vi "Dresden R2R Sputter 03.02.2018 IY24.vi"() -> ()   [LabVIEW 2009] (continued)
                        n3270 = local write "Pps_code_entry"("PF187=" ("Pps_code_entry")) -> ()
                      }
                      frame #1 {
                        n3271 = Wait (ms)(milliseconds to wait=u32 500) -> ()  [unwired: 1 out]
                      }
                      frame #2 {
                        n3272 = local write "Ppsok"(TRUE ("Ppsok")) -> ()
                      }
                    }
                  }
                }
              }
            }
            n3273 = case shown="True" w5019 {
              tunnel: w5023 -> [_ w5431]
              frame #0 {
              }
              frame #1 {
                n3274 = case shown="False" w5431 {
                  frame #0 {
                    n3275 = stacked-sequence {
                      frame #0 {
                        n3276 = local write "Pps_code_entry"("PF118=" ("Pps_code_entry")) -> ()
                      }
                      frame #1 {
                        n3277 = Wait (ms)(milliseconds to wait=u32 500) -> ()  [unwired: 1 out]
                      }
                      frame #2 {
                        n3278 = local write "Ppsok"(TRUE ("Ppsok")) -> ()
                      }
                    }
                  }
                  frame #1 {
                    n3279 = stacked-sequence {
                      frame #0 {
                        n3280 = local write "Pps_code_entry"("PF117=" ("Pps_code_entry")) -> ()
                      }
                      frame #1 {
                        n3281 = Wait (ms)(milliseconds to wait=u32 500) -> ()  [unwired: 1 out]
                      }
                      frame #2 {
                        n3282 = local write "Ppsok"(TRUE ("Ppsok")) -> ()
                      }
                    }
                  }
                }
              }
            }
            n3283 = case shown="True" w4829 {
              tunnel: w4833 -> [_ w5074]
              frame #0 {
              }
              frame #1 {
                n3284 = case shown="True" w5074 {
                  frame #0 {
                    n3285 = stacked-sequence {
                      frame #0 {
                        n3286 = local write "Pps_code_entry"("PF218=" ("Pps_code_entry")) -> ()
                      }
                      frame #1 {
                        n3287 = Wait (ms)(milliseconds to wait=u32 500) -> ()  [unwired: 1 out]
                      }
                      frame #2 {
                        n3288 = local write "Ppsok"(TRUE ("Ppsok")) -> ()
                      }
                    }
                  }
                  frame #1 {
                    n3289 = stacked-sequence {
                      frame #0 {
                        n3290 = local write "Pps_code_entry"("PF217=" ("Pps_code_entry")) -> ()
                      }
                      frame #1 {
                        n3291 = Wait (ms)(milliseconds to wait=u32 500) -> ()  [unwired: 1 out]
                      }
                      frame #2 {
                        n3292 = local write "Ppsok"(TRUE ("Ppsok")) -> ()
                      }
                    }
                  }
                }
              }
            }
            n3293 = case shown="True" w5059 {
              tunnel: w5063 -> [_ w5487]
              frame #0 {
              }
              frame #1 {
                n3294 = case shown="False" w5487 {
                  frame #0 {
                    n3295 = stacked-sequence {
                      frame #0 {
                        n3296 = local write "Pps_code_entry"("PF114=" ("Pps_code_entry")) -> ()
                      }
                      frame #1 {
                        n3297 = Wait (ms)(milliseconds to wait=u32 500) -> ()  [unwired: 1 out]
                      }
                      frame #2 {
                        n3298 = local write "Ppsok"(TRUE ("Ppsok")) -> ()
                      }
                    }
                  }
                  frame #1 {
                    n3299 = stacked-sequence {
                      frame #0 {
                        n3300 = local write "Pps_code_entry"("PF113=" ("Pps_code_entry")) -> ()
                      }
                      frame #1 {
                        n3301 = Wait (ms)(milliseconds to wait=u32 500) -> ()  [unwired: 1 out]
                      }
                      frame #2 {
                        n3302 = local write "Ppsok"(TRUE ("Ppsok")) -> ()
                      }
                    }
                  }
                }
              }
            }
            n3303 = case shown="True" w4989 {
              tunnel: w4993 -> [_ w5305]
              frame #0 {
              }
              frame #1 {
                n3304 = case shown="True" w5305 {
                  frame #0 {
                    n3305 = stacked-sequence {
                      frame #0 {
                        n3306 = local write "Pps_code_entry"("PF154=" ("Pps_code_entry")) -> ()
                      }
                      frame #1 {
                        n3307 = Wait (ms)(milliseconds to wait=u32 500) -> ()  [unwired: 1 out]
                      }
                      frame #2 {
                        n3308 = local write "Ppsok"(TRUE ("Ppsok")) -> ()
                      }
                    }
                  }
                  frame #1 {
                    n3309 = stacked-sequence {
                      frame #0 {
                        n3310 = local write "Pps_code_entry"("PF153=" ("Pps_code_entry")) -> ()
                      }
                      frame #1 {
                        n3311 = Wait (ms)(milliseconds to wait=u32 500) -> ()  [unwired: 1 out]
                      }
                      frame #2 {
                        n3312 = local write "Ppsok"(TRUE ("Ppsok")) -> ()
                      }
                    }
                  }
                }
              }
            }
            n3313 = case shown="True" w4888 {
              tunnel: w4884 -> [_ w5256]
              frame #0 {
              }
              frame #1 {
                n3314 = case shown="False" w5256 {
                  frame #0 {
                    n3315 = stacked-sequence {
                      frame #0 {
                        n3316 = local write "Pps_code_entry"("PF175=" ("Pps_code_entry")) -> ()
                      }
                      frame #1 {
                        n3317 = Wait (ms)(milliseconds to wait=u32 500) -> ()  [unwired: 1 out]
                      }
                      frame #2 {
                        n3318 = local write "Ppsok"(TRUE ("Ppsok")) -> ()
                      }
                    }
                  }
                  frame #1 {
                    n3319 = stacked-sequence {
                      frame #0 {
                        n3320 = local write "Pps_code_entry"("PF175=" ("Pps_code_entry")) -> ()
                      }
                      frame #1 {
                        n3321 = Wait (ms)(milliseconds to wait=u32 500) -> ()  [unwired: 1 out]
                      }
                      frame #2 {
                        n3322 = local write "Ppsok"(TRUE ("Ppsok")) -> ()
                      }
                    }
                  }
                }
              }
            }
            n3323 = case shown="True" w4913 {
              tunnel: w4909 -> [_ w5172]
              frame #0 {
              }
              frame #1 {
                n3324 = case shown="False" w5172 {
                  frame #0 {
                    n3325 = stacked-sequence {
                      frame #0 {
                        n3326 = local write "Pps_code_entry"("PF186=" ("Pps_code_entry")) -> ()
                      }
                      frame #1 {
                        n3327 = Wait (ms)(milliseconds to wait=u32 500) -> ()  [unwired: 1 out]
                      }
                      frame #2 {
                        n3328 = local write "Ppsok"(TRUE ("Ppsok")) -> ()
                      }
                    }
                  }
                  frame #1 {
                    n3329 = stacked-sequence {
                      frame #0 {
                        n3330 = local write "Pps_code_entry"("PF185=" ("Pps_code_entry")) -> ()
                      }
                      frame #1 {
                        n3331 = Wait (ms)(milliseconds to wait=u32 500) -> ()  [unwired: 1 out]
                      }
                      frame #2 {
                        n3332 = local write "Ppsok"(TRUE ("Ppsok")) -> ()
                      }
                    }
                  }
                }
              }
            }
            n3333 = case shown="True" w4868 {
              tunnel: w4864 -> [_ w5228]
              frame #0 {
              }
              frame #1 {
                n3334 = case shown="False" w5228 {
                  frame #0 {
                    n3335 = stacked-sequence {
                      frame #0 {
                        n3336 = local write "Pps_code_entry"("PF180=" ("Pps_code_entry")) -> ()
                      }
                      frame #1 {
                        n3337 = Wait (ms)(milliseconds to wait=u32 500) -> ()  [unwired: 1 out]
                      }
                      frame #2 {
                        n3338 = local write "Ppsok"(TRUE ("Ppsok")) -> ()
                      }
                    }
                  }
                  frame #1 {
                    n3339 = stacked-sequence {
                      frame #0 {
                        n3340 = local write "Pps_code_entry"("PF179=" ("Pps_code_entry")) -> ()
                      }
                      frame #1 {
                        n3341 = Wait (ms)(milliseconds to wait=u32 500) -> ()  [unwired: 1 out]
                      }
                      frame #2 {
                        n3342 = local write "Ppsok"(TRUE ("Ppsok")) -> ()
                      }
                    }
                  }
                }
              }
            }
            n3343 = case shown="True" w4779 {
              tunnel: w4783 -> [_ w5144]
              frame #0 {
              }
              frame #1 {
                n3344 = case shown="False" w5144 {
                  frame #0 {
                    n3345 = stacked-sequence {
                      frame #0 {
                        n3346 = local write "Pps_code_entry"("PF210=" ("Pps_code_entry")) -> ()
                      }
                      frame #1 {
                        n3347 = Wait (ms)(milliseconds to wait=u32 500) -> ()  [unwired: 1 out]
                      }
                      frame #2 {
                        n3348 = local write "Ppsok"(TRUE ("Ppsok")) -> ()
                      }
                    }
                  }
                  frame #1 {
                    n3349 = stacked-sequence {
                      frame #0 {
                        n3350 = local write "Pps_code_entry"("PF209=" ("Pps_code_entry")) -> ()
                      }
                      frame #1 {
                        n3351 = Wait (ms)(milliseconds to wait=u32 500) -> ()  [unwired: 1 out]
                      }
                      frame #2 {
                        n3352 = local write "Ppsok"(TRUE ("Ppsok")) -> ()
                      }
                    }
                  }
                }
              }
            }
            n3353 = case shown="True" w5008 {
              tunnel: w5004 -> [_ w5410]
              frame #0 {
              }
              frame #1 {
                n3354 = case shown="False" w5410 {
                  frame #0 {
                    n3355 = stacked-sequence {
                      frame #0 {
                        n3356 = local write "Pps_code_entry"("PF120=" ("Pps_code_entry")) -> ()
                      }
                      frame #1 {
                        n3357 = Wait (ms)(milliseconds to wait=u32 500) -> ()  [unwired: 1 out]
                      }
                      frame #2 {
                        n3358 = local write "Ppsok"(TRUE ("Ppsok")) -> ()
                      }
                    }
                  }
                  frame #1 {
                    n3359 = stacked-sequence {
                      frame #0 {
                        n3360 = local write "Pps_code_entry"("PF119=" ("Pps_code_entry")) -> ()
                      }
                      frame #1 {
                        n3361 = Wait (ms)(milliseconds to wait=u32 500) -> ()  [unwired: 1 out]
                      }
                      frame #2 {
                        n3362 = local write "Ppsok"(TRUE ("Ppsok")) -> ()
                      }
                    }
                  }
                }
              }
            }
            n3363 = case shown="True" w4939 {
              tunnel: w4943 -> [_ w5375]
              frame #0 {
              }
              frame #1 {
                n3364 = case shown="True" w5375 {
                  frame #0 {
                    n3365 = stacked-sequence {
                      frame #0 {
                        n3366 = local write "Pps_code_entry"("PF142=" ("Pps_code_entry")) -> ()
                      }
                      frame #1 {
                        n3367 = Wait (ms)(milliseconds to wait=u32 500) -> ()  [unwired: 1 out]
                      }
                      frame #2 {
                        n3368 = local write "Ppsok"(TRUE ("Ppsok")) -> ()
                      }
                    }
                  }
                  frame #1 {
                    n3369 = stacked-sequence {
                      frame #0 {
                        n3370 = local write "Pps_code_entry"("PF141=" ("Pps_code_entry")) -> ()
                      }
                      frame #1 {
                        n3371 = Wait (ms)(milliseconds to wait=u32 500) -> ()  [unwired: 1 out]
                      }
                      frame #2 {
                        n3372 = local write "Ppsok"(TRUE ("Ppsok")) -> ()
                      }
                    }
                  }
                }
              }
            }
            n3373 = case shown="True" w4914 {
              tunnel: w4918 -> [_ w5284]
              frame #0 {
              }
              frame #1 {
                n3374 = case shown="False" w5284 {
                  frame #0 {
                    n3375 = stacked-sequence {
                      frame #0 {
                        n3376 = local write "Pps_code_entry"("PF152=" ("Pps_code_entry")) -> ()
                      }
                      frame #1 {
                        n3377 = Wait (ms)(milliseconds to wait=u32 500) -> ()  [unwired: 1 out]
                      }
                      frame #2 {
                        n3378 = local write "Ppsok"(TRUE ("Ppsok")) -> ()
                      }
                    }
                  }
                  frame #1 {
                    n3379 = stacked-sequence {
                      frame #0 {
                        n3380 = local write "Pps_code_entry"("PF151=" ("Pps_code_entry")) -> ()
                      }
                      frame #1 {
                        n3381 = Wait (ms)(milliseconds to wait=u32 500) -> ()  [unwired: 1 out]
                      }
                      frame #2 {
                        n3382 = local write "Ppsok"(TRUE ("Ppsok")) -> ()
                      }
                    }
                  }
                }
              }
            }
            n3383 = case shown="True" w4799 {
              tunnel: w4803 -> [_ w5116]
              frame #0 {
              }
              frame #1 {
                n3384 = case shown="True" w5116 {
                  frame #0 {
                    n3385 = stacked-sequence {
                      frame #0 {
                        n3386 = local write "Pps_code_entry"("PF214=" ("Pps_code_entry")) -> ()
                      }
                      frame #1 {
                        n3387 = Wait (ms)(milliseconds to wait=u32 500) -> ()  [unwired: 1 out]
                      }
                      frame #2 {
                        n3388 = local write "Ppsok"(TRUE ("Ppsok")) -> ()
                      }
                    }
                  }
                  frame #1 {
                    n3389 = stacked-sequence {
                      frame #0 {
                        n3390 = local write "Pps_code_entry"("PF213=" ("Pps_code_entry")) -> ()
                      }
                      frame #1 {
                        n3391 = Wait (ms)(milliseconds to wait=u32 500) -> ()  [unwired: 1 out]
                      }
                      frame #2 {
                        n3392 = local write "Ppsok"(TRUE ("Ppsok")) -> ()
                      }
                    }
                  }
                }
              }
            }
            n3393 = case shown="True" w4959 {
              tunnel: w4963 -> [_ w5347]
              frame #0 {
              }
              frame #1 {
                n3394 = case shown="True" w5347 {
                  frame #0 {
                    n3395 = stacked-sequence {
                      frame #0 {
                        n3396 = local write "Pps_code_entry"("PF146=" ("Pps_code_entry")) -> ()
                      }
                      frame #1 {
                        n3397 = Wait (ms)(milliseconds to wait=u32 500) -> ()  [unwired: 1 out]
                      }
                      frame #2 {
                        n3398 = local write "Ppsok"(TRUE ("Ppsok")) -> ()
                      }
                    }
                  }
                  frame #1 {
                    n3399 = stacked-sequence {
                      frame #0 {
                        n3400 = local write "Pps_code_entry"("PF145=" ("Pps_code_entry")) -> ()
                      }
                      frame #1 {
                        n3401 = Wait (ms)(milliseconds to wait=u32 500) -> ()  [unwired: 1 out]
                      }
                      frame #2 {
                        n3402 = local write "Ppsok"(TRUE ("Ppsok")) -> ()
                      }
                    }
                  }
                }
              }
            }
            n3403 = case shown="True" w5058 {
              tunnel: w5054 -> [_ w5480]
              frame #0 {
              }
              frame #1 {
                n3404 = case shown="False" w5480 {
                  frame #0 {
                    n3405 = stacked-sequence {
                      frame #0 {
                        n3406 = local write "Pps_code_entry"("PF112=" ("Pps_code_entry")) -> ()
                      }
                      frame #1 {
                        n3407 = Wait (ms)(milliseconds to wait=u32 500) -> ()  [unwired: 1 out]
                      }
                      frame #2 {
                        n3408 = local write "Ppsok"(TRUE ("Ppsok")) -> ()
                      }
                    }
                  }
                  frame #1 {
                    n3409 = stacked-sequence {
                      frame #0 {
                        n3410 = local write "Pps_code_entry"("PF111=" ("Pps_code_entry")) -> ()
                      }
                      frame #1 {
                        n3411 = Wait (ms)(milliseconds to wait=u32 500) -> ()  [unwired: 1 out]
                      }
                      frame #2 {
                        n3412 = local write "Ppsok"(TRUE ("Ppsok")) -> ()
                      }
                    }
                  }
                }
              }
            }
            n3413 = case shown="True" w5038 {
              tunnel: w5034 -> [_ w5452]
              frame #0 {
              }
              frame #1 {
                n3414 = case shown="False" w5452 {
                  frame #0 {
                    n3415 = stacked-sequence {
                      frame #0 {
                        n3416 = local write "Pps_code_entry"("PF116=" ("Pps_code_entry")) -> ()
                      }
                      frame #1 {
                        n3417 = Wait (ms)(milliseconds to wait=u32 500) -> ()  [unwired: 1 out]
                      }
                      frame #2 {
                        n3418 = local write "Ppsok"(TRUE ("Ppsok")) -> ()
                      }
                    }
                  }
                  frame #1 {
                    n3419 = stacked-sequence {
                      frame #0 {
                        n3420 = local write "Pps_code_entry"("PF115=" ("Pps_code_entry")) -> ()
                      }
                      frame #1 {
                        n3421 = Wait (ms)(milliseconds to wait=u32 500) -> ()  [unwired: 1 out]
                      }
                      frame #2 {
                        n3422 = local write "Ppsok"(TRUE ("Ppsok")) -> ()
                      }
                    }
                  }
                }
              }
            }
            n3423 = local read "Trns_gv_2_3_on"() -> (w4994:bool)
            n3424 = local read "Ch3_Bg_bv_on"() -> (w4844:bool)
            n3425 = local read "Trns_gv_1_2_on"() -> (w5003:bool)
            n3426 = local read "Ch4_Bg_bv_on"() -> (w4823:bool)
            n3427 = local read "Ch2_Bg_bv_on"() -> (w4983:bool)
            n3428 = local read "Ch3_Ch_atm_on"() -> (w4879:bool)
            n3429 = local read "Ch4_Ch_atm_on"() -> (w4788:bool)
            n3430 = local read "Ch2_Ch_atm_on"() -> (w4948:bool)
            n3431 = local read "Ch1_Bg_bv_on"() -> (w5014:bool)
            n3432 = local read "Ch3_Ch_cc_on"() -> (w4878:bool)
            n3433 = local read "Ch4_Ch_cc_on"() -> (w4789:bool)
            n3434 = local read "Ch1_Ch_atm_on"() -> (w5049:bool)
            n3435 = local read "Ch2_Ch_cc_on"() -> (w4949:bool)
            n3436 = local read "Ch1_Ch_cc_on"() -> (w5048:bool)
            n3437 = local read "Ch3_Ch_pg_on"() -> (w4863:bool)
            n3438 = local read "Ch4_Ch_pg_on"() -> (w4804:bool)
            n3439 = local read "Ch2_Ch_pg_on"() -> (w4964:bool)
            n3440 = local read "Ch1_Ch_pg_on"() -> (w5033:bool)
            n3441 = feedback #98() -> (w4862:bool)  [unwired: 1 in]
            n3442 = feedback #99() -> (w4845:bool)  [unwired: 1 in]
            n3443 = feedback #100() -> (w4995:bool)  [unwired: 1 in]
            n3444 = feedback #101() -> (w4805:bool)  [unwired: 1 in]
            n3445 = feedback #102() -> (w4822:bool)  [unwired: 1 in]
            n3446 = feedback #103() -> (w4965:bool)  [unwired: 1 in]
            n3447 = feedback #104() -> (w4982:bool)  [unwired: 1 in]
            n3448 = feedback #105() -> (w5002:bool)  [unwired: 1 in]
            n3449 = feedback #106() -> (w5032:bool)  [unwired: 1 in]
            n3450 = feedback #107() -> (w5015:bool)  [unwired: 1 in]
            n3451 = feedback #108() -> (w4877:bool)  [unwired: 1 in]
            n3452 = feedback #109() -> (w4790:bool)  [unwired: 1 in]
            n3453 = feedback #110() -> (w4950:bool)  [unwired: 1 in]
            n3454 = feedback #111() -> (w4880:bool)  [unwired: 1 in]
            n3455 = feedback #112() -> (w4787:bool)  [unwired: 1 in]
            n3456 = feedback #113() -> (w4947:bool)  [unwired: 1 in]
            n3457 = feedback #114() -> (w5047:bool)  [unwired: 1 in]
            n3458 = feedback #115() -> (w5050:bool)  [unwired: 1 in]
            n3459 = Boolean To (0,1)(Boolean=w4863) -> (0, 1=w4861:i16)
            n3460 = Boolean To (0,1)(Boolean=w4862) -> (0, 1=w4860:i16)
            n3461 = Boolean To (0,1)(Boolean=w4844) -> (0, 1=w4846:i16)
            n3462 = Boolean To (0,1)(Boolean=w4845) -> (0, 1=w4847:i16)
            n3463 = Boolean To (0,1)(Boolean=w4994) -> (0, 1=w4996:i16)
            n3464 = Boolean To (0,1)(Boolean=w4995) -> (0, 1=w4997:i16)
            n3465 = Boolean To (0,1)(Boolean=w4804) -> (0, 1=w4806:i16)
            n3466 = Boolean To (0,1)(Boolean=w4805) -> (0, 1=w4807:i16)
            n3467 = Boolean To (0,1)(Boolean=w4823) -> (0, 1=w4821:i16)
            n3468 = Boolean To (0,1)(Boolean=w4822) -> (0, 1=w4820:i16)
            n3469 = Boolean To (0,1)(Boolean=w4964) -> (0, 1=w4966:i16)
            n3470 = Boolean To (0,1)(Boolean=w4965) -> (0, 1=w4967:i16)
            n3471 = Boolean To (0,1)(Boolean=w4983) -> (0, 1=w4981:i16)
            n3472 = Boolean To (0,1)(Boolean=w4982) -> (0, 1=w4980:i16)
            n3473 = Boolean To (0,1)(Boolean=w5003) -> (0, 1=w5001:i16)
            n3474 = Boolean To (0,1)(Boolean=w5002) -> (0, 1=w5000:i16)
            n3475 = Boolean To (0,1)(Boolean=w5033) -> (0, 1=w5031:i16)
            n3476 = Boolean To (0,1)(Boolean=w5032) -> (0, 1=w5030:i16)
            n3477 = Boolean To (0,1)(Boolean=w5014) -> (0, 1=w5016:i16)
            n3478 = Boolean To (0,1)(Boolean=w5015) -> (0, 1=w5017:i16)
            n3479 = Boolean To (0,1)(Boolean=w4878) -> (0, 1=w4876:i16)
            n3480 = Boolean To (0,1)(Boolean=w4877) -> (0, 1=w4875:i16)
            n3481 = Boolean To (0,1)(Boolean=w4789) -> (0, 1=w4791:i16)
            n3482 = Boolean To (0,1)(Boolean=w4790) -> (0, 1=w4792:i16)
            n3483 = Boolean To (0,1)(Boolean=w4949) -> (0, 1=w4951:i16)
            n3484 = Boolean To (0,1)(Boolean=w4950) -> (0, 1=w4952:i16)
            n3485 = Boolean To (0,1)(Boolean=w4879) -> (0, 1=w4881:i16)
            n3486 = Boolean To (0,1)(Boolean=w4880) -> (0, 1=w4882:i16)
            n3487 = Boolean To (0,1)(Boolean=w4788) -> (0, 1=w4786:i16)
            n3488 = Boolean To (0,1)(Boolean=w4787) -> (0, 1=w4785:i16)
            n3489 = Boolean To (0,1)(Boolean=w4948) -> (0, 1=w4946:i16)
            n3490 = Boolean To (0,1)(Boolean=w4947) -> (0, 1=w4945:i16)
            n3491 = Boolean To (0,1)(Boolean=w5048) -> (0, 1=w5046:i16)
            n3492 = Boolean To (0,1)(Boolean=w5047) -> (0, 1=w5045:i16)
            n3493 = Boolean To (0,1)(Boolean=w5049) -> (0, 1=w5051:i16)
            n3494 = Boolean To (0,1)(Boolean=w5050) -> (0, 1=w5052:i16)
            n3495 = Not Equal?(x=w4861, y=w4860) -> (x != y?=w4859:bool)
            n3496 = Not Equal?(x=w4846, y=w4847) -> (x != y?=w4848:bool)
            n3497 = Not Equal?(x=w4996, y=w4997) -> (x != y?=w4998:bool)
            n3498 = Not Equal?(x=w4806, y=w4807) -> (x != y?=w4808:bool)
            n3499 = Not Equal?(x=w4821, y=w4820) -> (x != y?=w4819:bool)
            n3500 = Not Equal?(x=w4966, y=w4967) -> (x != y?=w4968:bool)
            n3501 = Not Equal?(x=w4981, y=w4980) -> (x != y?=w4979:bool)
            n3502 = Not Equal?(x=w5001, y=w5000) -> (x != y?=w4999:bool)
            n3503 = Not Equal?(x=w5031, y=w5030) -> (x != y?=w5029:bool)
            n3504 = Not Equal?(x=w5016, y=w5017) -> (x != y?=w5018:bool)
            n3505 = Not Equal?(x=w4876, y=w4875) -> (x != y?=w4874:bool)
            n3506 = Not Equal?(x=w4791, y=w4792) -> (x != y?=w4793:bool)
            n3507 = Not Equal?(x=w4951, y=w4952) -> (x != y?=w4953:bool)
            n3508 = Not Equal?(x=w4881, y=w4882) -> (x != y?=w4883:bool)
            n3509 = Not Equal?(x=w4786, y=w4785) -> (x != y?=w4784:bool)
            n3510 = Not Equal?(x=w4946, y=w4945) -> (x != y?=w4944:bool)
            n3511 = Not Equal?(x=w5046, y=w5045) -> (x != y?=w5044:bool)
            n3512 = Not Equal?(x=w5051, y=w5052) -> (x != y?=w5053:bool)
            n3513 = case shown="True" w4859 {
              tunnel: w4863 -> [_ w5221]
              frame #0 {
              }
              frame #1 {
                n3514 = case shown="True" w5221 {
                  frame #0 {
                    n3515 = stacked-sequence {
                      frame #0 {
                        n3516 = local write "Pps_code_entry"("PF194=" ("Pps_code_entry")) -> ()
                      }
                      frame #1 {
                        n3517 = Wait (ms)(milliseconds to wait=u32 500) -> ()  [unwired: 1 out]
                      }
                      frame #2 {
                        n3518 = local write "Ppsok"(TRUE ("Ppsok")) -> ()
                      }
                    }
                  }
                  frame #1 {
                    n3519 = stacked-sequence {
                      frame #0 {
                        n3520 = local write "Pps_code_entry"("PF193=" ("Pps_code_entry")) -> ()
                      }
                      frame #1 {
                        n3521 = Wait (ms)(milliseconds to wait=u32 500) -> ()  [unwired: 1 out]
                      }
                      frame #2 {
                        n3522 = local write "Ppsok"(TRUE ("Ppsok")) -> ()
                      }
                    }
                  }
                }
              }
            }
            n3523 = case shown="True" w4848 {
              tunnel: w4844 -> [_ w5200]
              frame #0 {
              }
              frame #1 {
                n3524 = case shown="True" w5200 {
                  frame #0 {
                    n3525 = stacked-sequence {
                      frame #0 {
                        n3526 = local write "Pps_code_entry"("PF196=" ("Pps_code_entry")) -> ()
                      }
                      frame #1 {
                        n3527 = Wait (ms)(milliseconds to wait=u32 500) -> ()  [unwired: 1 out]
                      }
                      frame #2 {
                        n3528 = local write "Ppsok"(TRUE ("Ppsok")) -> ()
                      }
                    }
                  }
                  frame #1 {
                    n3529 = stacked-sequence {
                      frame #0 {
                        n3530 = local write "Pps_code_entry"("PF195=" ("Pps_code_entry")) -> ()
                      }
                      frame #1 {
                        n3531 = Wait (ms)(milliseconds to wait=u32 500) -> ()  [unwired: 1 out]
                      }
                      frame #2 {
                        n3532 = local write "Ppsok"(TRUE ("Ppsok")) -> ()
                      }
                    }
                  }
                }
              }
            }
            n3533 = case shown="True" w4998 {
              tunnel: w4994 -> [_ w5298]
              frame #0 {
              }
              frame #1 {
                n3534 = case shown="False" w5298 {
                  frame #0 {
                    n3535 = stacked-sequence {
                      frame #0 {
                        n3536 = local write "Pps_code_entry"("PF164=" ("Pps_code_entry")) -> ()
                      }
                      frame #1 {
                        n3537 = Wait (ms)(milliseconds to wait=u32 500) -> ()  [unwired: 1 out]
                      }
                      frame #2 {
                        n3538 = local write "Ppsok"(TRUE ("Ppsok")) -> ()
                      }
                    }
                  }
                  frame #1 {
                    n3539 = stacked-sequence {
                      frame #0 {
                        n3540 = local write "Pps_code_entry"("PF163=" ("Pps_code_entry")) -> ()
                      }
                      frame #1 {
                        n3541 = Wait (ms)(milliseconds to wait=u32 500) -> ()  [unwired: 1 out]
                      }
                      frame #2 {
                        n3542 = local write "Ppsok"(TRUE ("Ppsok")) -> ()
                      }
                    }
                  }
                }
              }
            }
            n3543 = case shown="True" w4808 {
              tunnel: w4804 -> [_ w5109]
              frame #0 {
              }
              frame #1 {
                n3544 = case shown="True" w5109 {
                  frame #0 {
                    n3545 = stacked-sequence {
                      frame #0 {
                        n3546 = local write "Pps_code_entry"("PF224=" ("Pps_code_entry")) -> ()
                      }
                      frame #1 {
                        n3547 = Wait (ms)(milliseconds to wait=u32 500) -> ()  [unwired: 1 out]
                      }
                      frame #2 {
                        n3548 = local write "Ppsok"(TRUE ("Ppsok")) -> ()
                      }
                    }
                  }
                  frame #1 {
                    n3549 = stacked-sequence {
                      frame #0 {
                        n3550 = local write "Pps_code_entry"("PF223=" ("Pps_code_entry")) -> ()
                      }
                      frame #1 {
                        n3551 = Wait (ms)(milliseconds to wait=u32 500) -> ()  [unwired: 1 out]
                      }
                      frame #2 {
                        n3552 = local write "Ppsok"(TRUE ("Ppsok")) -> ()
                      }
                    }
                  }
                }
              }
            }
            n3553 = case shown="True" w4819 {
              tunnel: w4823 -> [_ w5088]
              frame #0 {
              }
              frame #1 {
                n3554 = case shown="False" w5088 {
                  frame #0 {
                    n3555 = stacked-sequence {
                      frame #0 {
                        n3556 = local write "Pps_code_entry"("PF226=" ("Pps_code_entry")) -> ()
                      }
                      frame #1 {
                        n3557 = Wait (ms)(milliseconds to wait=u32 500) -> ()  [unwired: 1 out]
                      }
                      frame #2 {
                        n3558 = local write "Ppsok"(TRUE ("Ppsok")) -> ()
                      }
                    }
                  }
                  frame #1 {
                    n3559 = stacked-sequence {
                      frame #0 {
                        n3560 = local write "Pps_code_entry"("PF225=" ("Pps_code_entry")) -> ()
                      }
                      frame #1 {
                        n3561 = Wait (ms)(milliseconds to wait=u32 500) -> ()  [unwired: 1 out]
                      }
                      frame #2 {
                        n3562 = local write "Ppsok"(TRUE ("Ppsok")) -> ()
                      }
                    }
                  }
                }
              }
            }
            n3563 = case shown="True" w4968 {
              tunnel: w4964 -> [_ w5340]
              frame #0 {
              }
              frame #1 {
                n3564 = case shown="True" w5340 {
                  frame #0 {
                    n3565 = stacked-sequence {
                      frame #0 {
                        n3566 = local write "Pps_code_entry"("PF160=" ("Pps_code_entry")) -> ()
                      }
                      frame #1 {
                        n3567 = Wait (ms)(milliseconds to wait=u32 500) -> ()  [unwired: 1 out]
                      }
                      frame #2 {
                        n3568 = local write "Ppsok"(TRUE ("Ppsok")) -> ()
                      }
                    }
                  }
                  frame #1 {
                    n3569 = stacked-sequence {
                      frame #0 {
                        n3570 = local write "Pps_code_entry"("PF159=" ("Pps_code_entry")) -> ()
                      }
                      frame #1 {
                        n3571 = Wait (ms)(milliseconds to wait=u32 500) -> ()  [unwired: 1 out]
                      }
                      frame #2 {
                        n3572 = local write "Ppsok"(TRUE ("Ppsok")) -> ()
                      }
                    }
                  }
                }
              }
            }
            n3573 = case shown="True" w4979 {
              tunnel: w4983 -> [_ w5319]
              frame #0 {
              }
              frame #1 {
                n3574 = case shown="False" w5319 {
                  frame #0 {
                    n3575 = stacked-sequence {
                      frame #0 {
                        n3576 = local write "Pps_code_entry"("PF162=" ("Pps_code_entry")) -> ()
                      }
                      frame #1 {
                        n3577 = Wait (ms)(milliseconds to wait=u32 500) -> ()  [unwired: 1 out]
                      }
                      frame #2 {
                        n3578 = local write "Ppsok"(TRUE ("Ppsok")) -> ()
                      }
                    }
                  }
                  frame #1 {
                    n3579 = stacked-sequence {
                      frame #0 {
                        n3580 = local write "Pps_code_entry"("PF161=" ("Pps_code_entry")) -> ()
                      }
                      frame #1 {
                        n3581 = Wait (ms)(milliseconds to wait=u32 500) -> ()  [unwired: 1 out]
                      }
                      frame #2 {
                        n3582 = local write "Ppsok"(TRUE ("Ppsok")) -> ()
                      }
                    }
                  }
                }
              }
            }
            n3583 = case shown="True" w4999 {
              tunnel: w5003 -> [_ w5403]
              frame #0 {
              }
              frame #1 {
                n3584 = case shown="True" w5403 {
                  frame #0 {
                    n3585 = stacked-sequence {
                      frame #0 {
                        n3586 = local write "Pps_code_entry"("PF130=" ("Pps_code_entry")) -> ()
                      }
                      frame #1 {
                        n3587 = Wait (ms)(milliseconds to wait=u32 500) -> ()  [unwired: 1 out]
                      }
                      frame #2 {
                        n3588 = local write "Ppsok"(TRUE ("Ppsok")) -> ()
                      }
                    }
                  }
                  frame #1 {
                    n3589 = stacked-sequence {
                      frame #0 {
                        n3590 = local write "Pps_code_entry"("PF129=" ("Pps_code_entry")) -> ()
                      }
                      frame #1 {
                        n3591 = Wait (ms)(milliseconds to wait=u32 500) -> ()  [unwired: 1 out]
                      }
                      frame #2 {
                        n3592 = local write "Ppsok"(TRUE ("Ppsok")) -> ()
                      }
                    }
                  }
                }
              }
            }
            n3593 = case shown="True" w5029 {
              tunnel: w5033 -> [_ w5445]
              frame #0 {
              }
              frame #1 {
                n3594 = case shown="False" w5445 {
                  frame #0 {
                    n3595 = stacked-sequence {
                      frame #0 {
                        n3596 = local write "Pps_code_entry"("PF126=" ("Pps_code_entry")) -> ()
                      }
                      frame #1 {
                        n3597 = Wait (ms)(milliseconds to wait=u32 500) -> ()  [unwired: 1 out]
                      }
                      frame #2 {
                        n3598 = local write "Ppsok"(TRUE ("Ppsok")) -> ()
                      }
                    }
                  }
                  frame #1 {
                    n3599 = stacked-sequence {
                      frame #0 {
                        n3600 = local write "Pps_code_entry"("PF125=" ("Pps_code_entry")) -> ()
                      }
                      frame #1 {
                        n3601 = Wait (ms)(milliseconds to wait=u32 500) -> ()  [unwired: 1 out]
                      }
                      frame #2 {
                        n3602 = local write "Ppsok"(TRUE ("Ppsok")) -> ()
                      }
                    }
                  }
                }
              }
            }
            n3603 = case shown="True" w5018 {
              tunnel: w5014 -> [_ w5424]
              frame #0 {
              }
              frame #1 {
                n3604 = case shown="True" w5424 {
                  frame #0 {
                    n3605 = stacked-sequence {
                      frame #0 {
                        n3606 = local write "Pps_code_entry"("PF128=" ("Pps_code_entry")) -> ()
                      }
                      frame #1 {
                        n3607 = Wait (ms)(milliseconds to wait=u32 500) -> ()  [unwired: 1 out]
                      }
                      frame #2 {
                        n3608 = local write "Ppsok"(TRUE ("Ppsok")) -> ()
                      }
                    }
                  }
                  frame #1 {
                    n3609 = stacked-sequence {
                      frame #0 {
                        n3610 = local write "Pps_code_entry"("PF127=" ("Pps_code_entry")) -> ()
                      }
                      frame #1 {
                        n3611 = Wait (ms)(milliseconds to wait=u32 500) -> ()  [unwired: 1 out]
                      }
                      frame #2 {
                        n3612 = local write "Ppsok"(TRUE ("Ppsok")) -> ()
                      }
                    }
                  }
                }
              }
            }
            n3613 = case shown="True" w4874 {
              tunnel: w4878 -> [_ w5242]
              frame #0 {
              }
              frame #1 {
                n3614 = case shown="False" w5242 {
                  frame #0 {
                    n3615 = stacked-sequence {
                      frame #0 {
                        n3616 = local write "Pps_code_entry"("PF192=" ("Pps_code_entry")) -> ()
                      }
                      frame #1 {
                        n3617 = Wait (ms)(milliseconds to wait=u32 500) -> ()  [unwired: 1 out]
                      }
                      frame #2 {
                        n3618 = local write "Ppsok"(TRUE ("Ppsok")) -> ()
                      }
                    }
                  }
                  frame #1 {
                    n3619 = stacked-sequence {
                      frame #0 {
                        n3620 = local write "Pps_code_entry"("PF191=" ("Pps_code_entry")) -> ()
                      }
                      frame #1 {
                        n3621 = Wait (ms)(milliseconds to wait=u32 500) -> ()  [unwired: 1 out]
                      }
                      frame #2 {
                        n3622 = local write "Ppsok"(TRUE ("Ppsok")) -> ()
                      }
                    }
                  }
                }
              }
            }
            n3623 = case shown="True" w4793 {
              tunnel: w4789 -> [_ w5130]
              frame #0 {
              }
              frame #1 {
                n3624 = case shown="False" w5130 {
                  frame #0 {
                    n3625 = stacked-sequence {
                      frame #0 {
                        n3626 = local write "Pps_code_entry"("PF222=" ("Pps_code_entry")) -> ()
                      }
                      frame #1 {
                        n3627 = Wait (ms)(milliseconds to wait=u32 500) -> ()  [unwired: 1 out]
                      }
                      frame #2 {
                        n3628 = local write "Ppsok"(TRUE ("Ppsok")) -> ()
                      }
                    }
                  }
                  frame #1 {
                    n3629 = stacked-sequence {
                      frame #0 {
                        n3630 = local write "Pps_code_entry"("PF221=" ("Pps_code_entry")) -> ()
                      }
                      frame #1 {
                        n3631 = Wait (ms)(milliseconds to wait=u32 500) -> ()  [unwired: 1 out]
                      }
                      frame #2 {
                        n3632 = local write "Ppsok"(TRUE ("Ppsok")) -> ()
                      }
                    }
                  }
                }
              }
            }
            n3633 = case shown="True" w4953 {
              tunnel: w4949 -> [_ w5361]
              frame #0 {
              }
              frame #1 {
                n3634 = case shown="True" w5361 {
                  frame #0 {
                    n3635 = stacked-sequence {
                      frame #0 {
                        n3636 = local write "Pps_code_entry"("PF158=" ("Pps_code_entry")) -> ()
                      }
                      frame #1 {
                        n3637 = Wait (ms)(milliseconds to wait=u32 500) -> ()  [unwired: 1 out]
                      }
                      frame #2 {
                        n3638 = local write "Ppsok"(TRUE ("Ppsok")) -> ()
                      }
                    }
                  }
                  frame #1 {
                    n3639 = stacked-sequence {
                      frame #0 {
                        n3640 = local write "Pps_code_entry"("PF157=" ("Pps_code_entry")) -> ()
                      }
                      frame #1 {
                        n3641 = Wait (ms)(milliseconds to wait=u32 500) -> ()  [unwired: 1 out]
                      }
                      frame #2 {
                        n3642 = local write "Ppsok"(TRUE ("Ppsok")) -> ()
                      }
                    }
                  }
                }
              }
            }
            n3643 = case shown="True" w4883 {
              tunnel: w4879 -> [_ w5249]
              frame #0 {
              }
              frame #1 {
                n3644 = case shown="False" w5249 {